vi "Main.vi"() -> ()   [LabVIEW 2018]
doc: "This template is for the Queued Message Handler design pattern.\n\nThe Event Handling Loop generates messages based on user interface actions.\n\nThe Message Handling Loop processes messages generated by the Event Handling Loop, or by other messages. The messages are string values, so new messages can be added easily to the Message Cases case structure in the Message Handling Loop. Each message cluster can also provide an optional value for Message Data, which is a variant that can be converted to whatever message-specific data is required."
uses:
  controls/UI Data.ctl
  <vilib>/Utility/miscctls.llb/LVPointDoubleTypeDef.ctl
  support/Message Queue/Enqueue Message (Single).vi
  <vilib>/Utility/error.llb/Error Cluster From Error Code.vi
  <vilib>/ErrorRing/Error Ring.xnode
  support/Message Queue/Message Queue.lvlib
  support/User Event - Stop/User Event - Stop.lvlib
panel:
  in  "X Scale.Offset and Multiplier:Offset":dbl
  out "XY Graph":cluster{dbl[], dbl[]}[](graph)
  out "Display <Replace Me>":string
  in  "Do Something Else <Replace Me>":bool
  in  "Do Something <Replace Me>":bool
  in  "Exit":bool
  # "This template is for the Queued Message Handler design pattern.\n\nSee the block diagram for more information on how to use this template."
  # "These controls have associated \"Value Changed\" events configured in the Event Structure on the diagram.\n\nReplace them (and reconfigure the Event Structure) with the controls you need for your application."
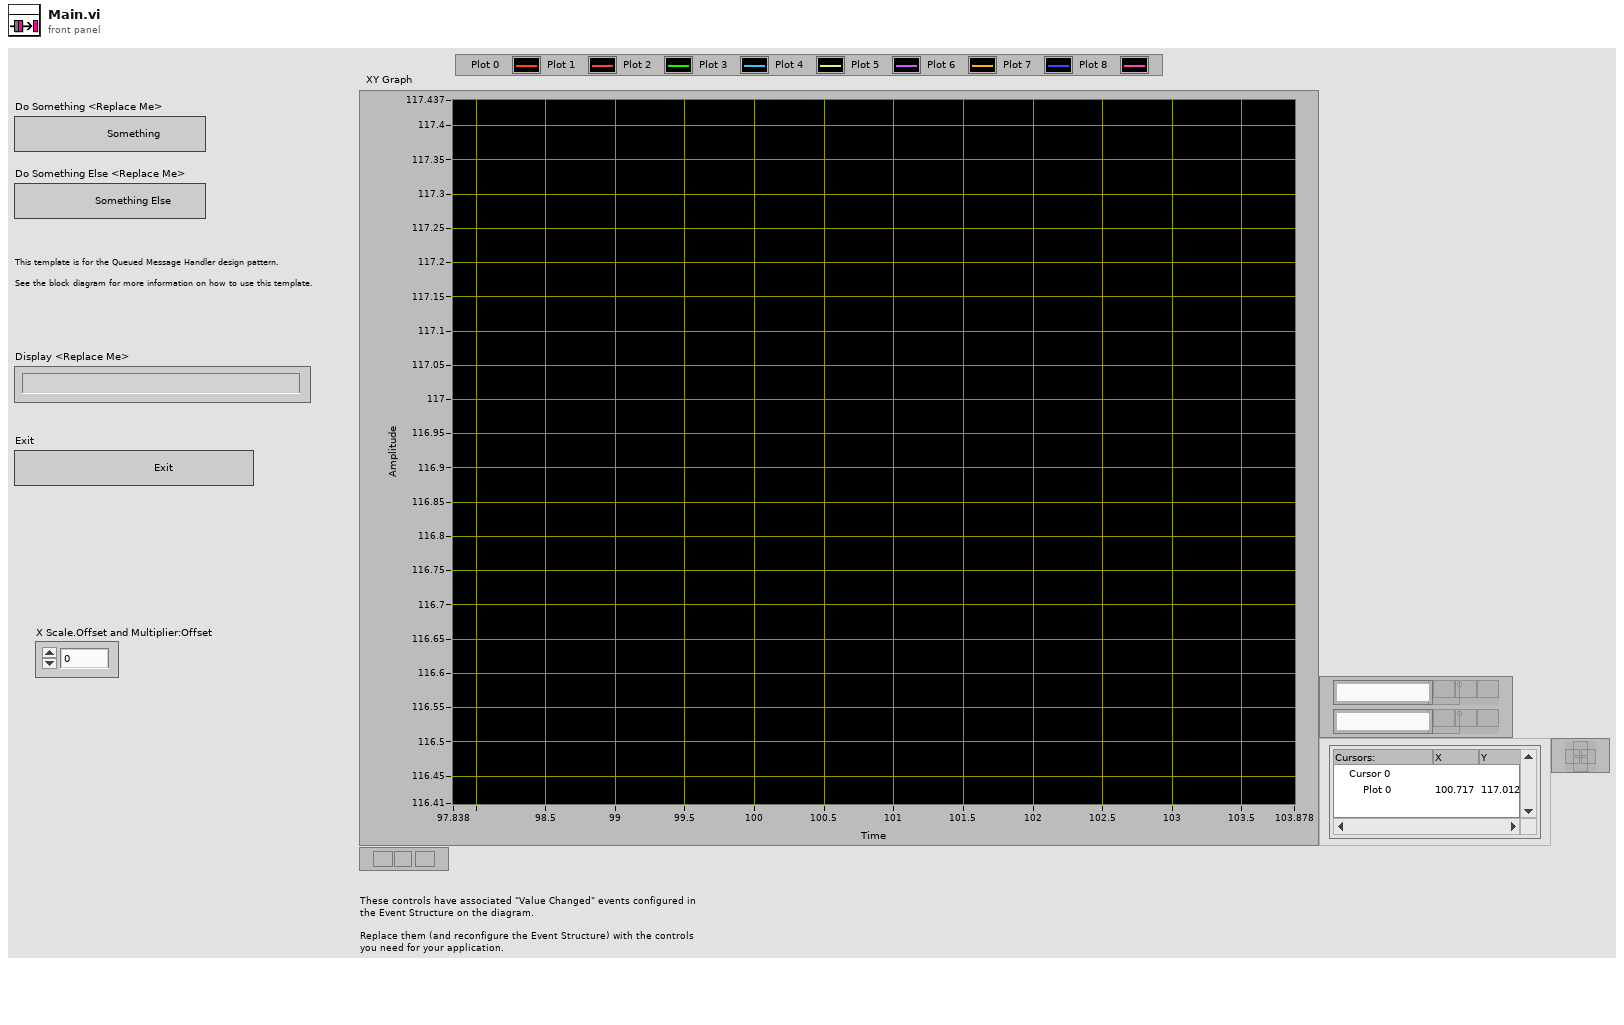
[diagram p1: front panel]
types:
  T1 = typedef "UI Data.ctl" = cluster{"Boolean <Replace Me>":bool, "String <Replace Me>":string, "Numeric <Replace Me>":dbl, "Do Something Ref":refnum<vi>, "Do Something Else Ref":refnum<vi>, "Data Display Ref":refnum<vi>, "Exit Button Ref":refnum<vi>, "CAD_Data":cluster{dbl[], dbl[]}[], "Reference":cluster{"XY Graph":refnum<vi>}}
  T2 = typedef "Message Queue.lvlib/All Message Queues.ctl" = cluster{"UI":refnum<queue>}
  T3 = typedef "LVPointDoubleTypeDef.ctl" = cluster{"X":dbl, "Y":dbl}
  T4 = cluster{"Name":string, "Color":u32, "Style":u8, "Point Style":u8, "Name Visible":bool, "Allow Drag":bool, "Annotation Mode":u32, "Plot":i32, "Index":i32, "Position":cluster{"X":dbl, "Y":dbl}, "X Scale":u32, "Y Scale":u32, "Show Arrow":bool, "Lock Name":bool, "Plot Area":i32, "Label Offset":cluster{"X":dbl, "Y":dbl}}
  T5 = typedef "LVPoint32TypeDef.ctl" = cluster{"Horizontal":i32, "Vertical":i32}
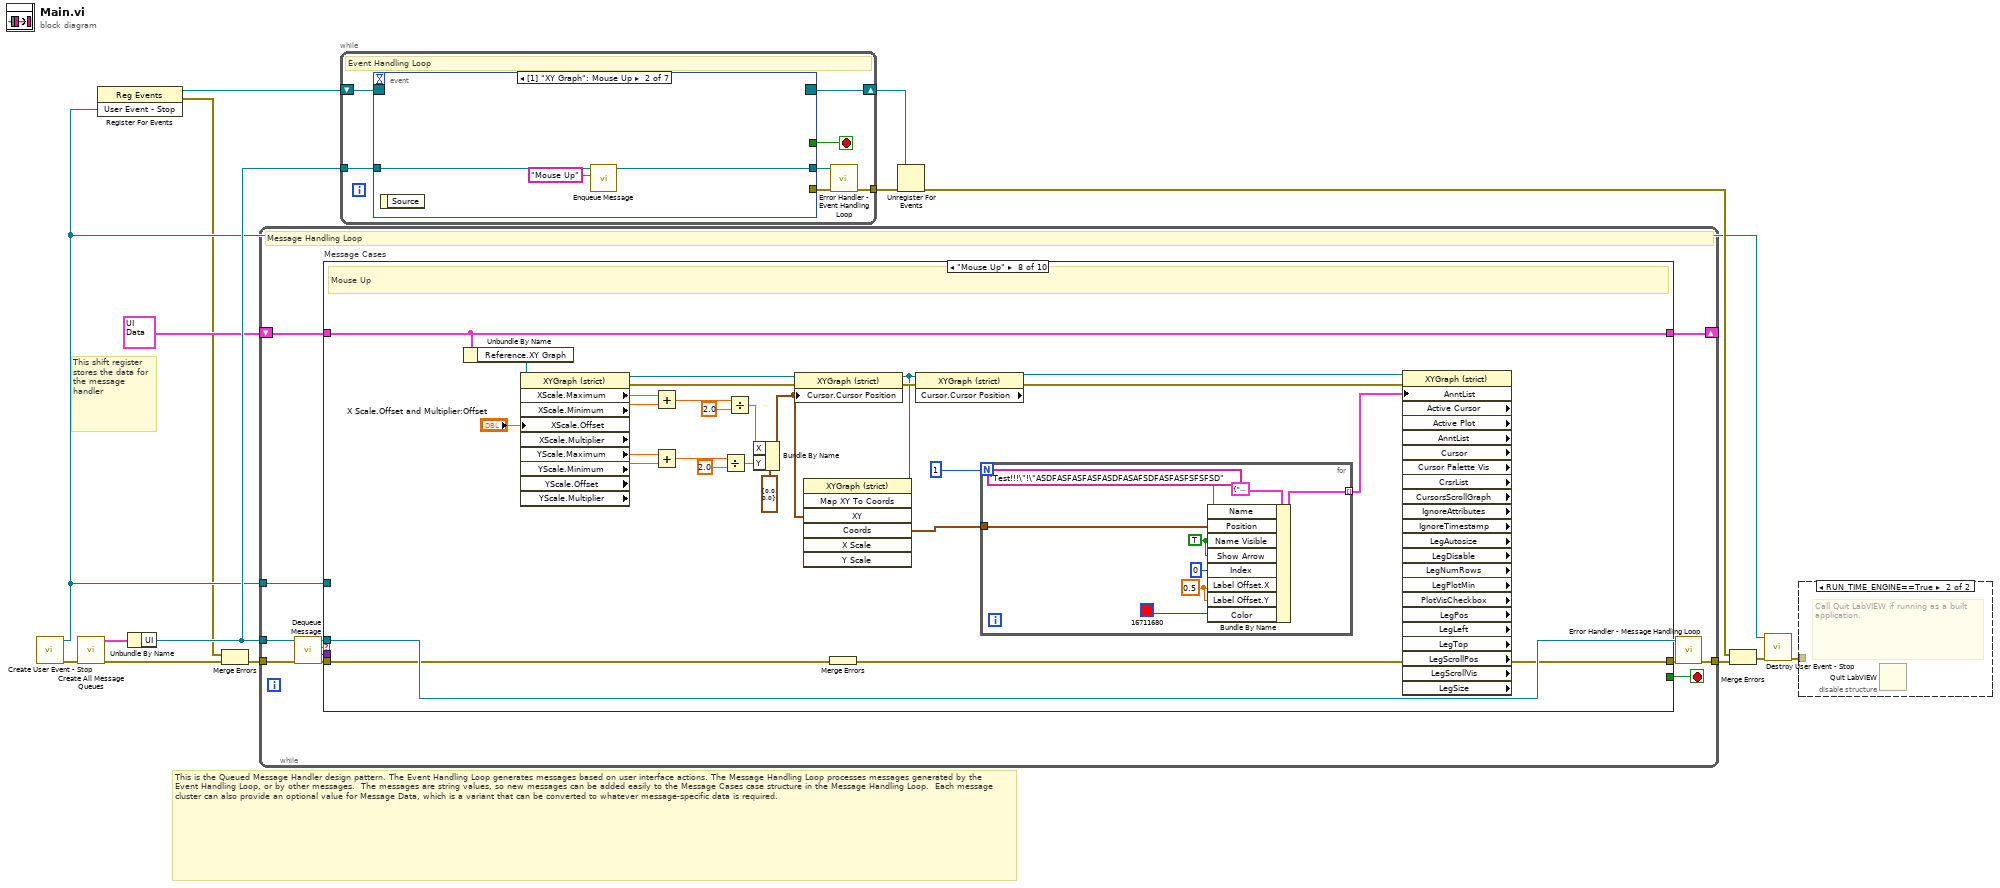
[diagram p0: block diagram]
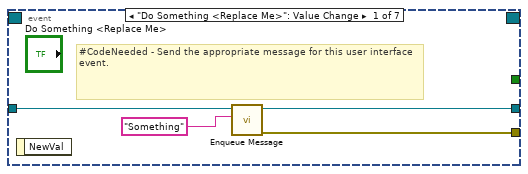
[diagram p3: hidden frame]
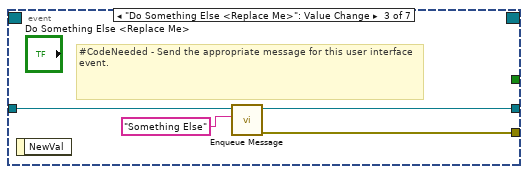
[diagram p4: hidden frame]
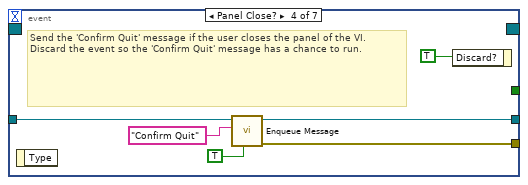
[diagram p5: hidden frame]
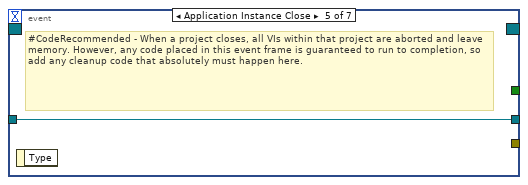
[diagram p6: hidden frame]
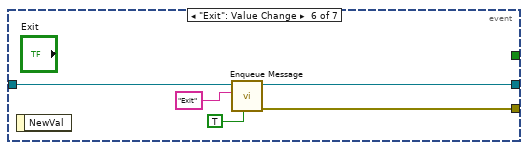
[diagram p7: hidden frame]
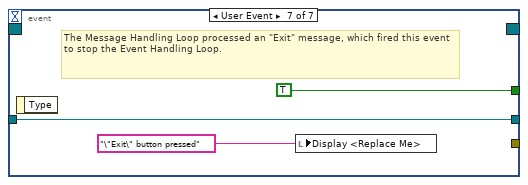
[diagram p8: hidden frame]
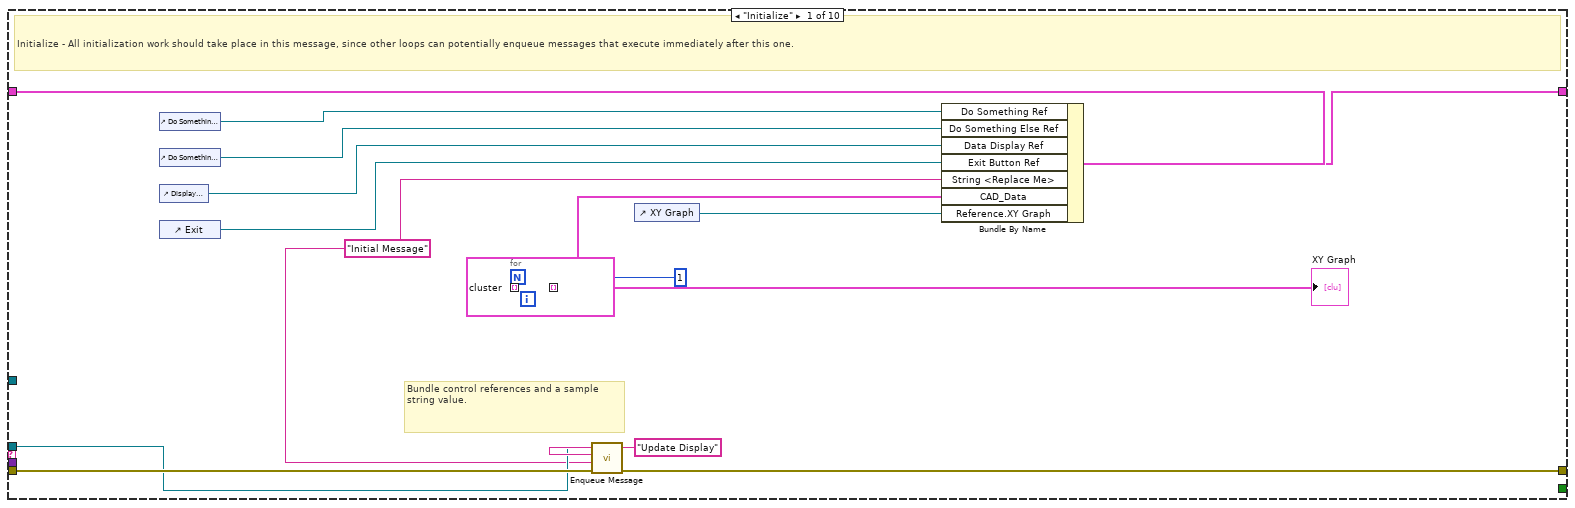
[diagram p9: hidden frame]
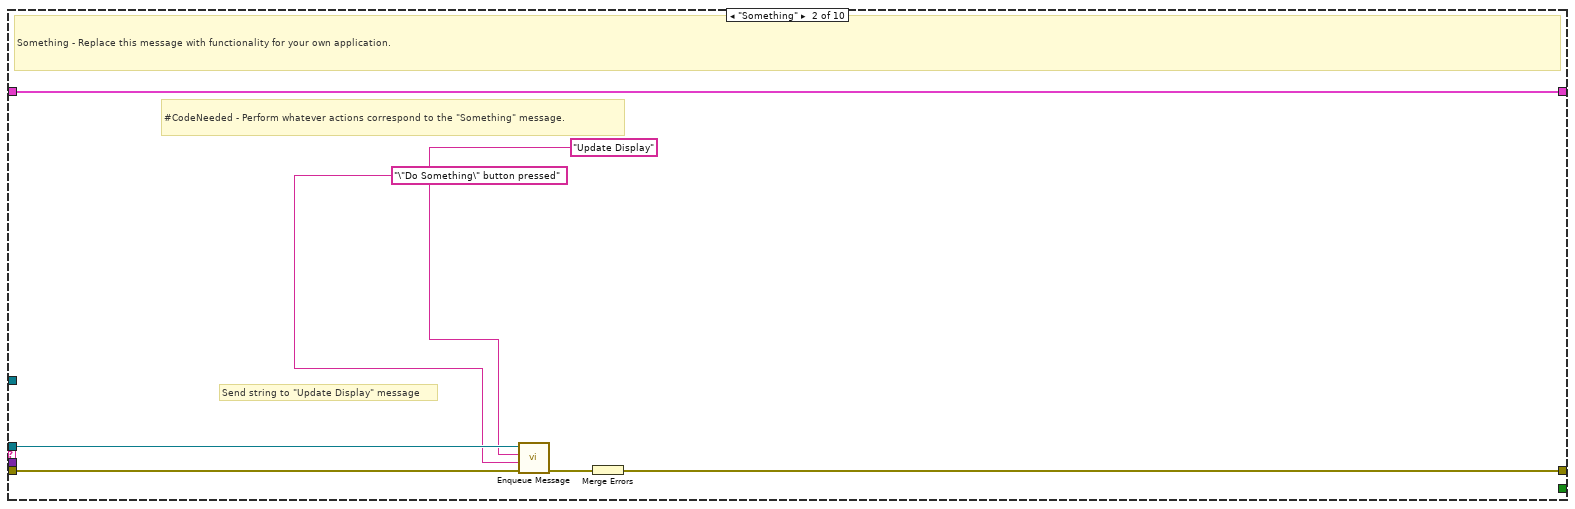
[diagram p10: hidden frame]
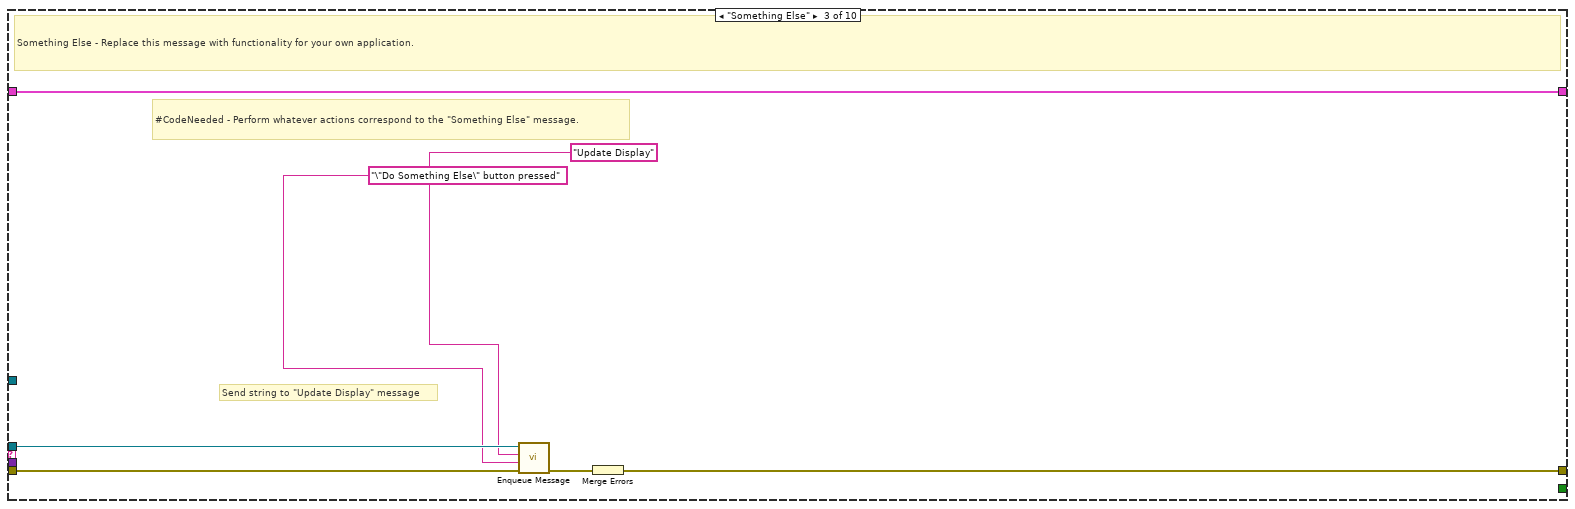
[diagram p11: hidden frame]
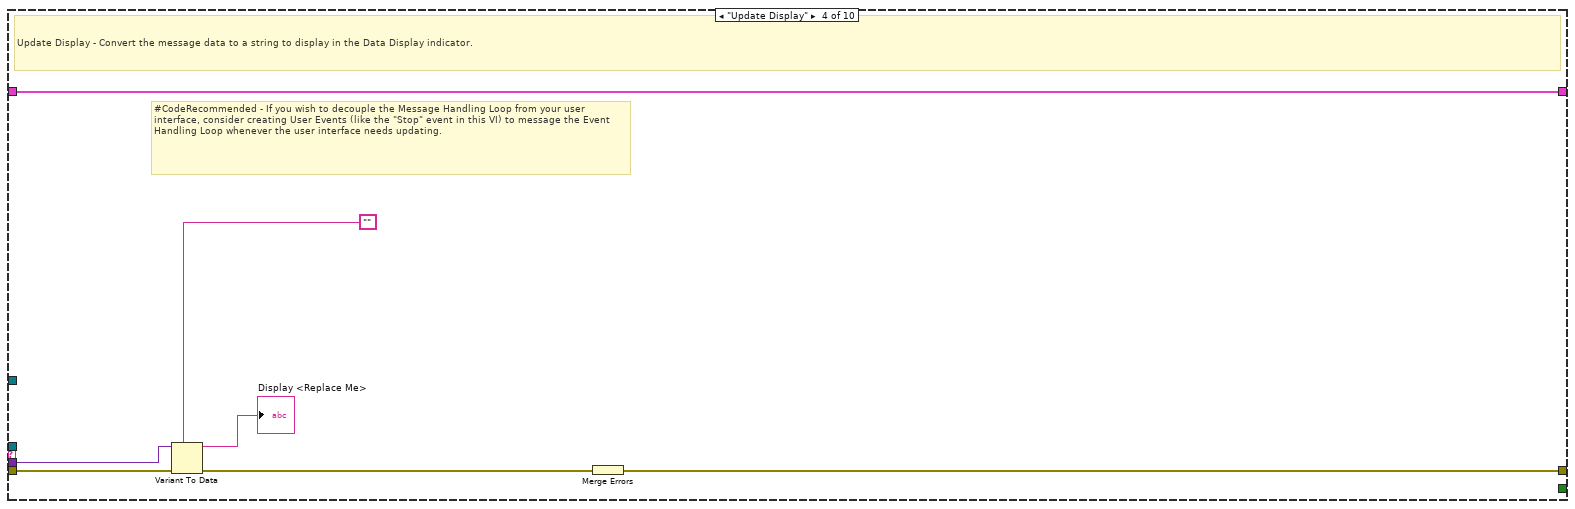
[diagram p12: hidden frame]
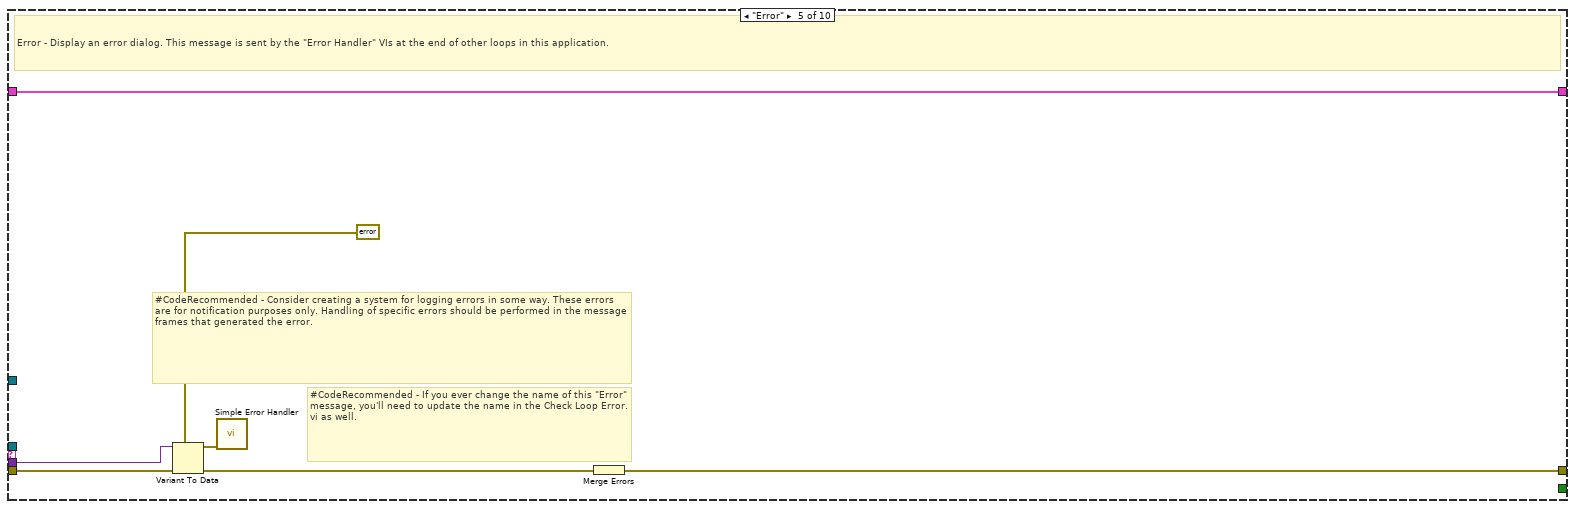
[diagram p13: hidden frame]
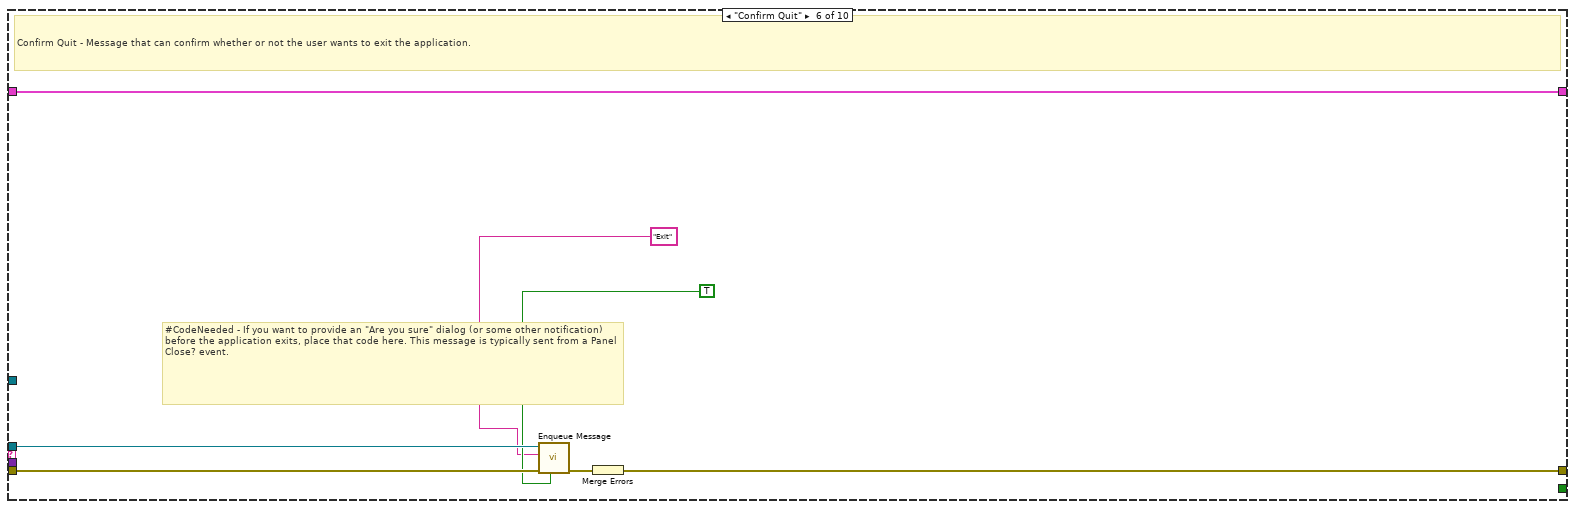
[diagram p14: hidden frame]
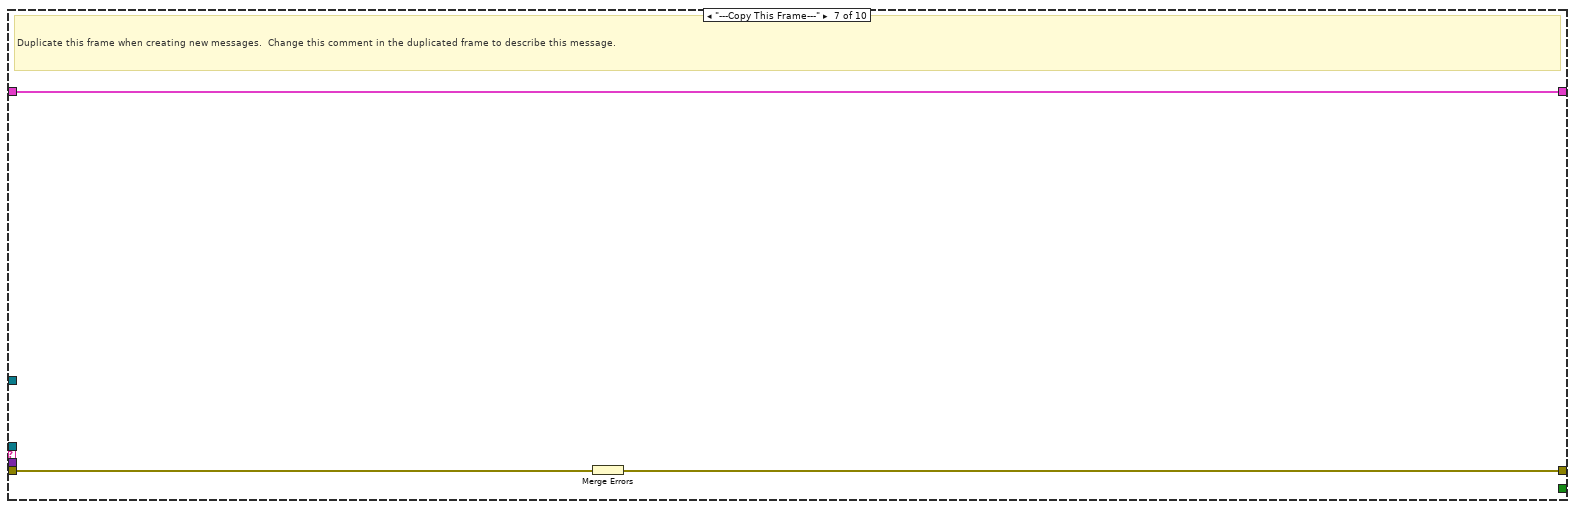
[diagram p15: hidden frame]
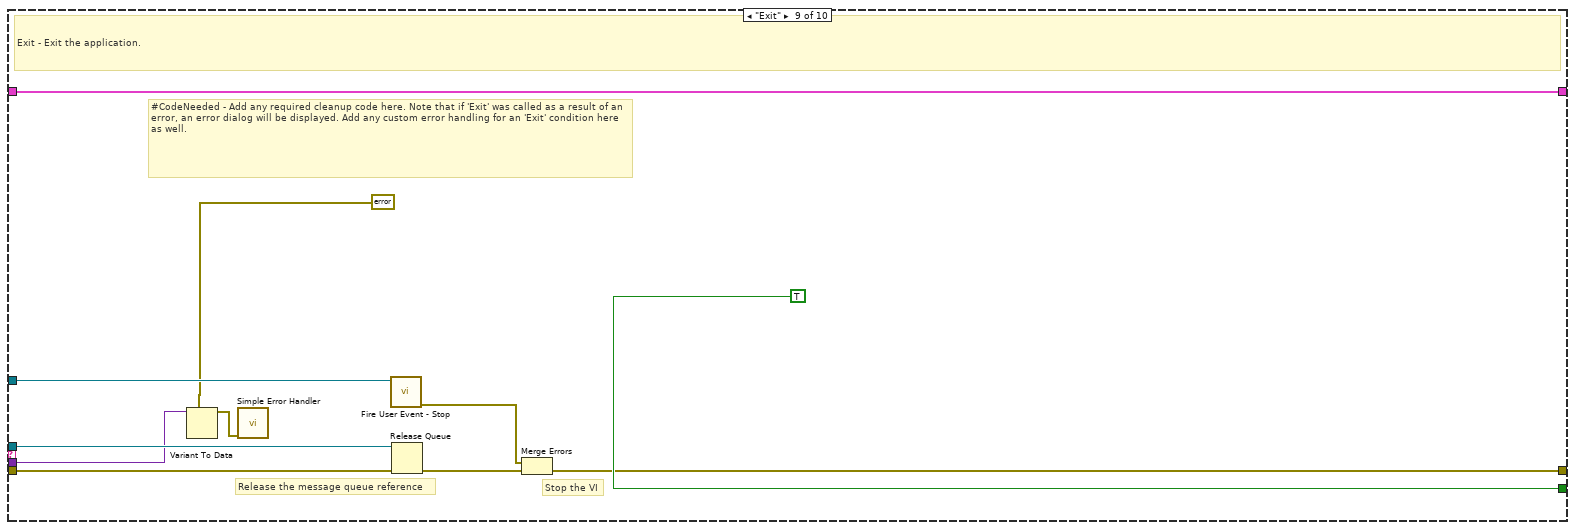
[diagram p16: hidden frame]
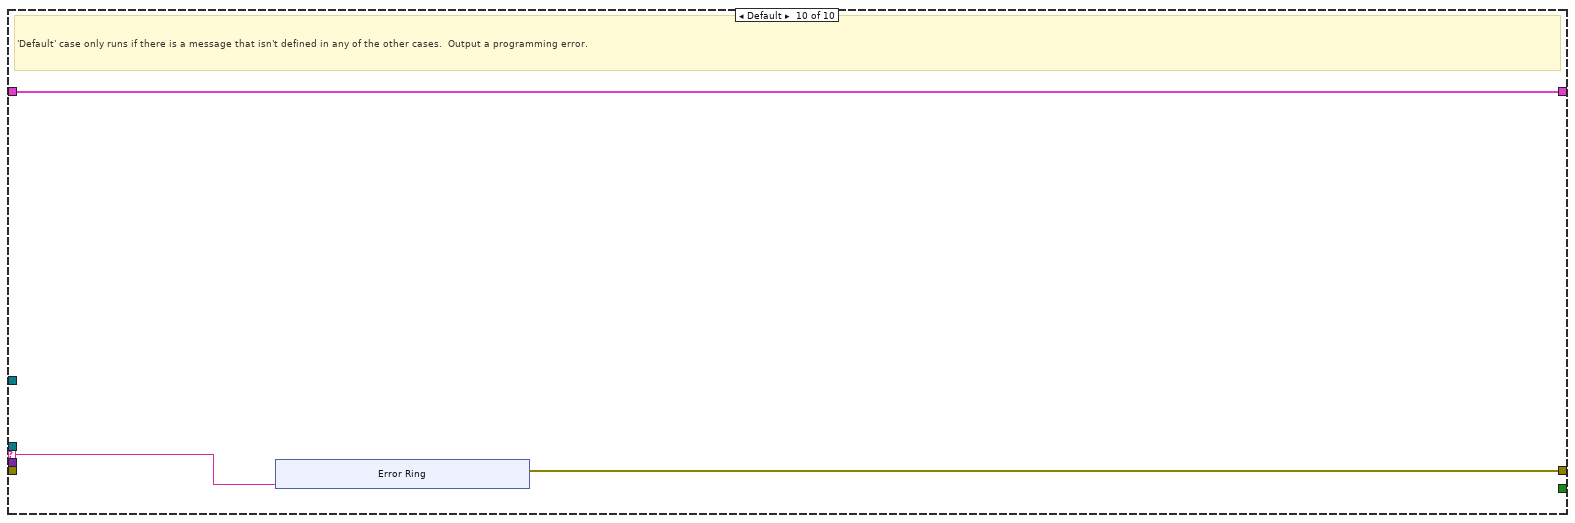
[diagram p17: hidden frame]
diagram:
  # "This is the Queued Message Handler design pattern. The Event Handling Loop generates messages based on user interface actions. The Message Handling Loop processes messages generated by the Event Handling Loop, or by other messages.  The messages are string values, so new messages can be added easily to the Message Cases case structure in the Message Handling Loop.  Each message cluster can also provide an optional value for Message Data, which is a variant that can be converted to whatever message-specific data is required."
  # "This shift register stores the data for the message handler"
  n1 = call "Create User Event - Stop.vi"() -> ("error out"=w11:errorcluster, "User Event - Stop"=w3:refnum<user-event>)  [unwired: 10 in]
  n2 = call "Create All Message Queues.vi"("error in (no error)"=w11) -> ("error out"=w15:errorcluster, "Message Queues out"=w14:T2)  [unwired: 9 in]
  n3 = register-events(w3) -> (reference out=w4:refnum<event-registration>, error out=w1:errorcluster)  [unwired: 2 in]
  n4 = Unbundle By Name(w14) -> ("UI"=w12:refnum<queue>)
  n5 = Merge Errors(w1, w15) -> (w2:errorcluster)
  n6 = while {
    tunnel: w12 -> [w19]
    shift-right: [w26] -> _
    shift-left: T1 {"Boolean <Replace Me>"=FALSE, "String <Replace Me>"="", "Numeric <Replace Me>"=0.0, "Do Something Ref"=refnum, "Do Something Else Ref"=refnum, "Data Display Ref"=refnum, "Exit Button Ref"=refnum, "CAD_Data"=[{array[1801 elements], array[1801 elements]}, {array[46807 elements], array[46807 elements]}, {array[492003 elements], array[492003 elements]}, {array[314618 elements], array[314618 elements]}, {array[31626 elements], array[31626 elements]}, {array[569211 elements], array[569211 elements]}], "Reference"={"XY Graph"=refnum}} ("Data Cluster") -> [w27]
    tunnel: w3 -> [w24]
    tunnel: w2 -> [w23]
    tunnel: [w17] -> w13
    stop <- w25 stop-if-true
    # "Message Handling Loop"
    n7 = call "Dequeue Message.vi"("error in (no error)"=w23, "Message Queue"=w19) -> ("error out"=w22:errorcluster, "Message Data"=w20:variant, "Message"=w21:string, "dup Message Queue"=w18:refnum<queue>)  [unwired: 6 in]
    n8 = case "Message Cases" shown="\"Mouse Up\"" w21 {
      selector: w21 -> [_ _ _ _ _ _ _ _ _ w127]
      tunnel: w18 -> [w33 w46 w53 _ _ w74 _ _ w126 _]
      tunnel: w22 -> [w41 w48 w55 w62 w71 w78 w81 w107 w119 _]
      tunnel: [w42 w49 w56 w63 w65 w76 w79 w106 w122 w128] -> w16
      tunnel: w27 -> [w40 w50 w57 w64 w70 w77 w80 w105 w125 w129]
      tunnel: [w39 w50 w57 w64 w70 w77 w80 w105 w125 w129] -> w26
      tunnel: [_ _ _ _ _ _ _ _ TRUE _] -> w25
      tunnel: w20 -> [_ _ _ w61 w69 _ _ _ w116 _]
      tunnel: w24 -> [_ _ _ _ _ _ _ _ w121 _]
      frame "Initialize" {
        w32 = "Initial Message" ("Initial Message")
        # "Bundle control references and a sample string value."
        # "Initialize - All initialization work should take place in this message, since other loops can potentially enqueue messages that execute immediately after this one."
        n9 = control-ref of="Do Something <Replace Me>"() -> (w38:refnum<vi>)
        n10 = control-ref of="Do Something Else <Replace Me>"() -> (w37:refnum<vi>)
        n11 = control-ref of="Display <Replace Me>"() -> (w36:refnum<vi>)
        n12 = control-ref of="Exit"() -> (w35:refnum<vi>)
        n13 = for {
          N: 1 -> [_]
          tunnel: cluster{dbl[], dbl[]}[] [{array[1801 elements], array[1801 elements]}, {array[46807 elements], array[46807 elements]}, {array[492003 elements], array[492003 elements]}, {array[314618 elements], array[314618 elements]}, {array[31626 elements], array[31626 elements]}, {array[569211 elements], array[569211 elements]}] ("Value") -> [w43] mode=indexing
          tunnel: [w43] -> w30 mode=indexing
        }
        "XY Graph" <- w30
        n14 = call-poly "Enqueue Message.vi"("error in (no error)"=w41, "Message Data"=w32, "Message"="Update Display", "Message Queue"=w33) -> ("error out"=w42:errorcluster)  [unwired: 6 in, 1 out]
        n15 = control-ref of="XY Graph"() -> (w28:refnum<vi>)
        n16 = Bundle By Name(cluster=w40, "Do Something Ref"=w38, "Do Something Else Ref"=w37, "Data Display Ref"=w36, "Exit Button Ref"=w35, "String <Replace Me>"=w32, "CAD_Data"=w30, "Reference.XY Graph"=w28) -> (w39:T1)
      }
      frame "Something" {
        # "Send string to \"Update Display\" message"
        # "#CodeNeeded - Perform whatever actions correspond to the \"Something\" message."
        # "Something - Replace this message with functionality for your own application."
        n17 = call-poly "Enqueue Message.vi"("error in (no error)"=w48, "Message Data"="\"Do Something\" button pressed" ("\"Do Something\" button pressed"), "Message"="Update Display", "Message Queue"=w46) -> ("error out"=w47:errorcluster)  [unwired: 6 in, 1 out]
        n18 = Merge Errors(w47) -> (w49:errorcluster)
      }
      frame "Something Else" {
        # "Send string to \"Update Display\" message"
        # "#CodeNeeded - Perform whatever actions correspond to the \"Something Else\" message."
        # "Something Else - Replace this message with functionality for your own application."
        n19 = call-poly "Enqueue Message.vi"("error in (no error)"=w55, "Message Data"="\"Do Something Else\" button pressed" ("\"Do Something Else\" button pressed"), "Message"="Update Display", "Message Queue"=w53) -> ("error out"=w54:errorcluster)  [unwired: 6 in, 1 out]
        n20 = Merge Errors(w54) -> (w56:errorcluster)
      }
      frame "Update Display" {
        # "#CodeRecommended - If you wish to decouple the Message Handling Loop from your user interface, consider creating User Events (like the \"Stop\" event in this VI) to message the Event Handling Loop whenever the user interface needs updating."
        # "Update Display - Convert the message data to a string to display in the Data Display indicator."
        n21 = Variant To Data(error in=w62, type="", Variant=w61) -> (data=→"Display <Replace Me>":string, error out=w59:errorcluster)
        n22 = Merge Errors(w59) -> (w63:errorcluster)
      }
      frame "Error" {
        # "#CodeRecommended - If you ever change the name of this \"Error\" message, you'll need to update the name in the Check Loop Error.vi as well."
        # "#CodeRecommended - Consider creating a system for logging errors in some way. These errors are for notification purposes only. Handling of specific errors should be performed in the message frames that generated the error."
        # "Error - Display an error dialog. This message is sent by the \"Error Handler\" VIs at the end of other loops in this application."
        n23 = Variant To Data(error in=w71, type=errorcluster {"status"=FALSE, "code"=0, "source"=""} ("error constant"), Variant=w69) -> (data=w67:errorcluster, error out=w66:errorcluster)
        n24 = call <vilib>:"Simple Error Handler.vi"("error in (no error)"=w67) -> ()  [unwired: 4 in, 5 out]
        n25 = Merge Errors(w66) -> (w65:errorcluster)
      }
      frame "Confirm Quit" {
        # "#CodeNeeded - If you want to provide an \"Are you sure\" dialog (or some other notification) before the application exits, place that code here. This message is typically sent from a Panel Close? event."
        # "Confirm Quit - Message that can confirm whether or not the user wants to exit the application."
        n26 = call-poly "Enqueue Message.vi"("Priority Message? (F)"=TRUE, "error in (no error)"=w78, "Message"="Exit", "Message Queue"=w74) -> ("error out"=w75:errorcluster)  [unwired: 6 in, 1 out]
        n27 = Merge Errors(w75) -> (w76:errorcluster)
      }
      frame "---Copy This Frame---" {
        # "Duplicate this frame when creating new messages.  Change this comment in the duplicated frame to describe this message."
        n28 = Merge Errors(w81) -> (w79:errorcluster)
      }
      frame "Mouse Up" {
        # "Mouse Up"
        n29 = Unbundle By Name(w105) -> ("Reference.XY Graph"=w104:refnum<vi>)
        n30 = property class="XYGraph (strict)" props=["XScale", "Maximum", "XScale", "Minimum", "XScale", "Offset", "XScale", "Multiplier", "YScale", "Maximum", "YScale", "Minimum", "YScale", "Offset", "YScale", "Multiplier"](reference=w104, "XScale.Offset"="X Scale.Offset and Multiplier:Offset") -> (reference out=w103:refnum<vi>, error out=w87:errorcluster, "XScale.Maximum"=w102:dbl, "XScale.Minimum"=w101:dbl, "YScale.Maximum"=w100:dbl, "YScale.Minimum"=w99:dbl)  [unwired: 1 in, 3 out]
        n31 = Add(x=w102, y=w101) -> (x+y=w98:dbl)
        n32 = Add(x=w100, y=w99) -> (x+y=w97:dbl)
        n33 = Divide(x=w97, y=2.0) -> (x/y=w92:dbl)
        n34 = Divide(x=w98, y=2.0) -> (x/y=w93:dbl)
        n35 = Bundle By Name(cluster=T3 {"X"=0.0, "Y"=0.0} ("Cursor.Cursor Position"), "X"=w93, "Y"=w92) -> (w83:T3)
        n36 = property class="XYGraph (strict)"(reference=w103, error in=w87, "Cursor.Cursor Position"=w83) -> (reference out=w84:refnum<vi>, error out=w86:errorcluster)
        n37 = invoke class="XYGraph (strict)" method="Map XY To Coords"(reference=w84, "XY"=w83) -> ("Coords"=w82:T5)  [unwired: 5 in, 6 out]
        n38 = Merge Errors(w107) -> (w106:errorcluster)
        n39 = property class="XYGraph (strict)" props=["Cursor", "Cursor Position"](reference=w84, error in=w86) -> (reference out=w89:refnum<vi>, error out=w85:errorcluster)  [unwired: 1 out]
        n40 = for {
          N: 1 -> [_]
          tunnel: [w115] -> w88 mode=indexing
          tunnel: w82 -> [w108]
          w110 = 0.5 ("Label Offset.X")
          w112 = TRUE ("Name Visible")
          n41 = Bundle By Name(cluster=T4 {"Name"="", "Color"=0, "Style"=0, "Point Style"=0, "Name Visible"=FALSE, "Allow Drag"=FALSE, "Annotation Mode"=0, "Plot"=0, "Index"=0, "Position"={"X"=0.0, "Y"=0.0}, "X Scale"=0, "Y Scale"=0, "Show Arrow"=FALSE, "Lock Name"=FALSE, "Plot Area"=0, "Label Offset"={"X"=0.0, "Y"=0.0}}, "Name"="Test!!!\"!\"ASDFASFASFASFASDFASAFSDFASFASFSFSFSD", "Position"=w108, "Name Visible"=w112, "Show Arrow"=w112, "Index"=0, "Label Offset.X"=w110, "Label Offset.Y"=w110, "Color"=u32 16711680) -> (w115:T4)
        }
        n42 = property class="XYGraph (strict)" props=["AnntList", "Active Cursor", "Active Plot", "AnntList", "Cursor", "Cursor Palette Vis", "CrsrList", "CursorsScrollGraph", "IgnoreAttributes", "IgnoreTimestamp", "LegAutosize", "LegDisable", "LegNumRows", "LegPlotMin", "PlotVisCheckbox", "LegPos", "LegLeft", "LegTop", "LegScrollPos", "LegScrollVis", "LegSize"](reference=w89, error in=w85, "AnntList"=w88) -> ()  [unwired: 22 out]
      }
      frame "Exit" {
        # "Stop the VI"
        # "Release the message queue reference"
        # "#CodeNeeded - Add any required cleanup code here. Note that if 'Exit' was called as a result of an error, an error dialog will be displayed. Add any custom error handling for an 'Exit' condition here as well."
        # "Exit - Exit the application."
        n43 = Variant To Data(type=errorcluster {"status"=FALSE, "code"=0, "source"=""} ("error constant"), Variant=w116) -> (data=w117:errorcluster)  [unwired: 1 in, 1 out]
        n44 = call <vilib>:"Simple Error Handler.vi"("error in (no error)"=w117) -> ()  [unwired: 4 in, 5 out]
        n45 = call "Fire User Event - Stop.vi"("User Event - Stop"=w121) -> ("error out"=w120:errorcluster)  [unwired: 10 in]
        n46 = Release Queue(queue=w126, error in (no error)=w119) -> (error out=w123:errorcluster)  [unwired: 1 in, 2 out]
        n47 = Merge Errors(w120, w123) -> (w122:errorcluster)
      }
      frame Default {
        # "'Default' case only runs if there is a message that isn't defined in any of the other cases.  Output a programming error."
        n48 = xnode "Error Ring"("parameter 0"=w127) -> ("error out"=w128:errorcluster)
      }
    }
    n49 = call "Error Handler - Message Handling Loop.vi"("error in (no error)"=w16, "Message Queue"=w18) -> ("dup error in"=w17:errorcluster)  [unwired: 8 in, 1 out]
  }
  n50 = while {
    tunnel: w12 -> [w143]
    shift-right: [w141] -> w8
    shift-left: w4 -> [w142]
    tunnel: [w137] -> w5
    stop <- w139 stop-if-true
    # "Event Handling Loop"
    n51 = event shown="[1] \"XY Graph\": Mouse Up" {
      selector: w142 -> [_ _ _ _ _ _ _]
      dyn-events: [_ _ _ _ _ _ _] -> w141
      timeout: _ -> [_ _ _ _ _ _ _]
      tunnel: [_ _ _ _ _ _ TRUE ("Discard?")] -> w139
      tunnel: w143 -> [w147 w150 w154 w159 w161 w166 w169]
      tunnel: [w144 _ w151 w158 _ w165 _] -> w140
      tunnel: [w146 w149 w153 w157 w161 w164 w169] -> w138
      event "Do Something <Replace Me>": Value Change {
        # "#CodeNeeded - Send the appropriate message for this user interface event."
        n52 = event-data() -> ()  [unwired: 1 in, 1 out]
        n53 = call-poly "Enqueue Message.vi"("Message"="Something", "Message Queue"=w147) -> ("error out"=w144:errorcluster, "dup Message Queue"=w146:refnum<queue>)  [unwired: 8 in]
      }
      event "XY Graph": Mouse Up {
        n54 = event-data() -> ()  [unwired: 1 in, 1 out]
        n55 = call-poly "Enqueue Message.vi"("Message"="Mouse Up", "Message Queue"=w150) -> ("dup Message Queue"=w149:refnum<queue>)  [unwired: 8 in, 1 out]
      }
      event "Do Something Else <Replace Me>": Value Change {
        # "#CodeNeeded - Send the appropriate message for this user interface event."
        n56 = event-data() -> ()  [unwired: 1 in, 1 out]
        n57 = call-poly "Enqueue Message.vi"("Message"="Something Else", "Message Queue"=w154) -> ("error out"=w151:errorcluster, "dup Message Queue"=w153:refnum<queue>)  [unwired: 8 in]
      }
      event Panel Close? {
        # "Send the 'Confirm Quit' message if the user closes the panel of the VI. Discard the event so the 'Confirm Quit' message has a chance to run."
        n58 = event-data() -> ()  [unwired: 1 in, 1 out]
        n59 = call-poly "Enqueue Message.vi"("Priority Message? (F)"=TRUE, "Message"="Confirm Quit", "Message Queue"=w159) -> ("error out"=w158:errorcluster, "dup Message Queue"=w157:refnum<queue>)  [unwired: 7 in]
        n60 = event-data("Discard?"=TRUE) -> ()  [unwired: 1 in, 1 out]
      }
      event Application Instance Close {
        # "#CodeRecommended - When a project closes, all VIs within that project are aborted and leave memory. However, any code placed in this event frame is guaranteed to run to completion, so add any cleanup code that absolutely must happen here."
        n61 = event-data() -> ()  [unwired: 1 in, 1 out]
      }
      event "Exit": Value Change {
        n62 = event-data() -> ()  [unwired: 1 in, 1 out]
        n63 = call-poly "Enqueue Message.vi"("Priority Message? (F)"=TRUE, "Message"="Exit", "Message Queue"=w166) -> ("error out"=w165:errorcluster, "dup Message Queue"=w164:refnum<queue>)  [unwired: 7 in]
      }
      event User Event {
        # "The Message Handling Loop processed an \"Exit\" message, which fired this event to stop the Event Handling Loop."
        n64 = event-data() -> ()  [unwired: 1 in, 1 out]
        n65 = local write "Display <Replace Me>"("\"Exit\" button pressed" ("VI Stopped")) -> ()
      }
    }
    n66 = call "Error Handler - Event Handling Loop.vi"("error in (no error)"=w140, "Message Queue"=w138) -> ("dup error in"=w137:errorcluster)  [unwired: 8 in, 1 out]
  }
  n67 = Unregister For Events(event registration refnum=w8, error in=w5) -> (error out=w9:errorcluster)
  n68 = Merge Errors(w9, w13) -> (w10:errorcluster)
  n69 = call "Destroy User Event - Stop.vi"("error in (no error)"=w10, "User Event - Stop"=w3) -> ("error out"=w6:errorcluster)  [unwired: 9 in]
  n70 = disable-structure shown="RUN_TIME_ENGINE==True" {
    disable-tunnel: w6 -> [_ _]
    frame condition #0 (active) {
    }
    frame condition #1 {
      # "Call Quit LabVIEW if running as a built application."
      n71 = Quit LabVIEW() -> ()  [unwired: 1 in]
    }
  }
